vi "ScanDelay_FTIR_PointSpectroscopy.vi"() -> ()   [LabVIEW 2022 SP3] (continued)
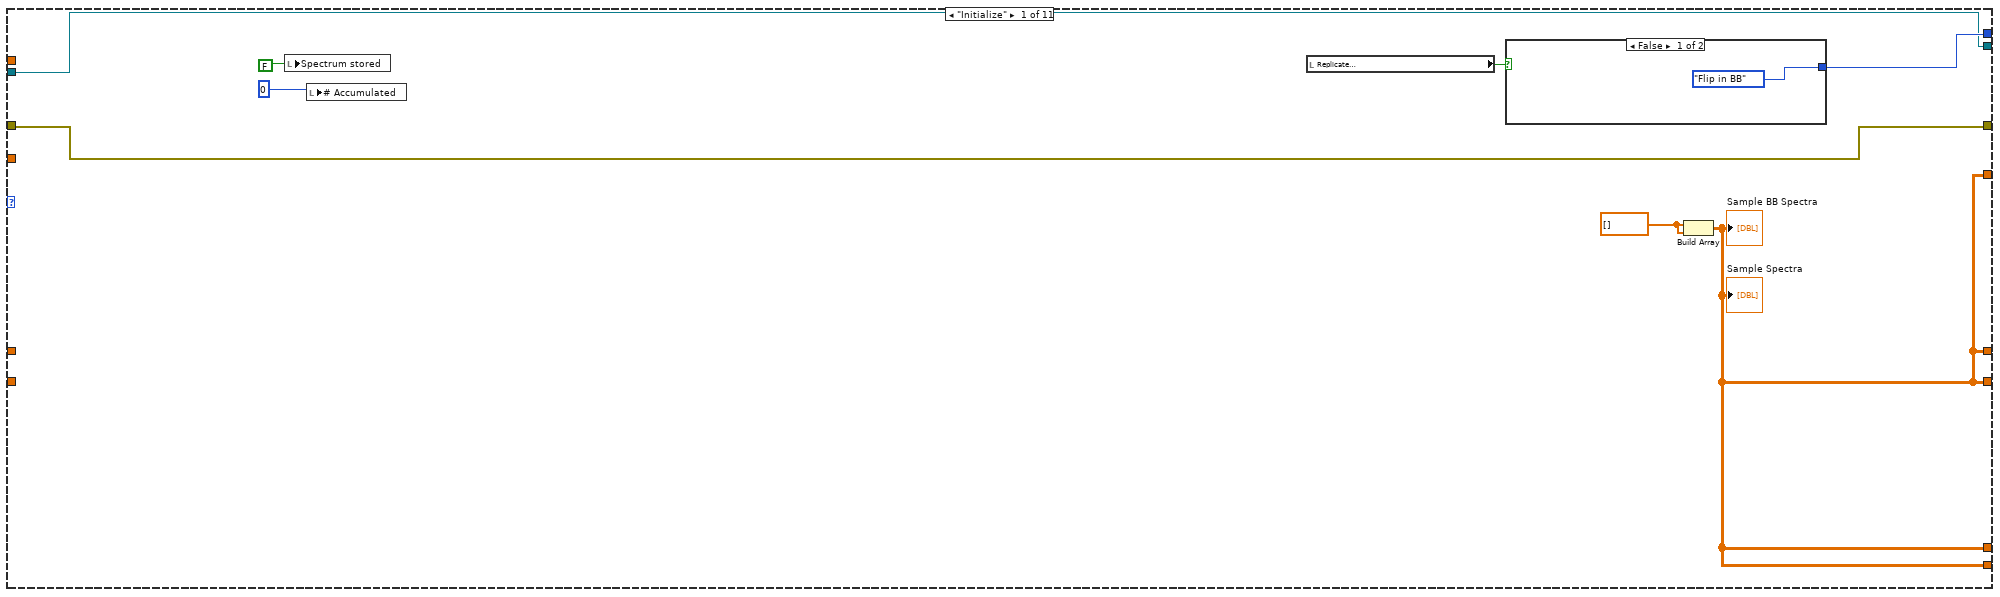
[diagram p3: hidden frame]
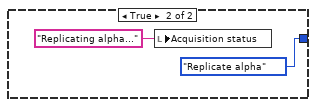
[diagram p4: hidden frame]
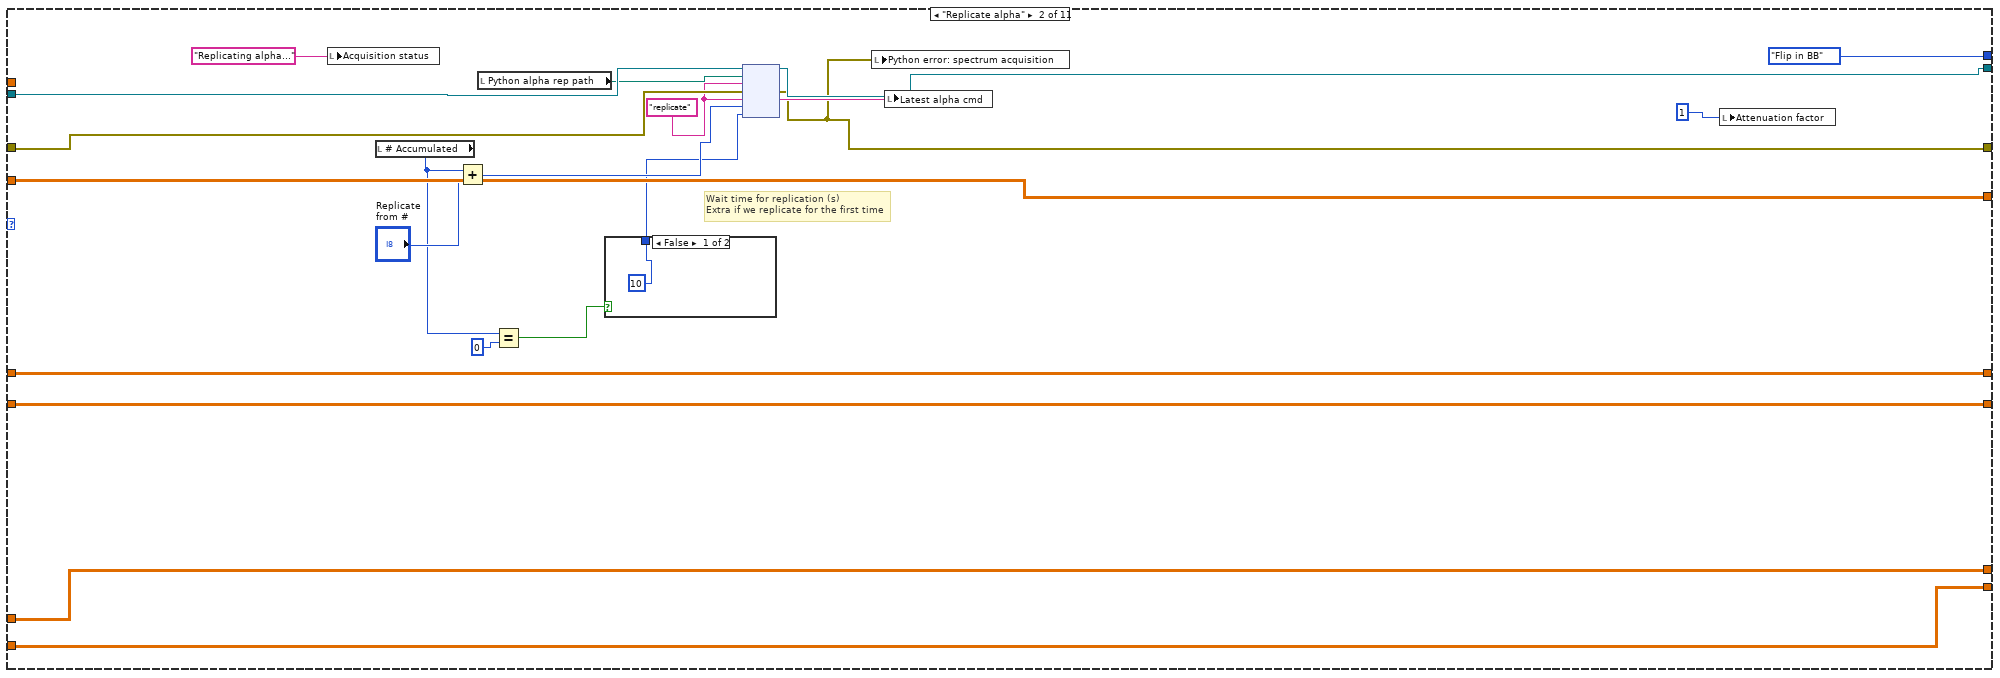
[diagram p5: hidden frame]
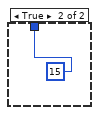
[diagram p6: hidden frame]
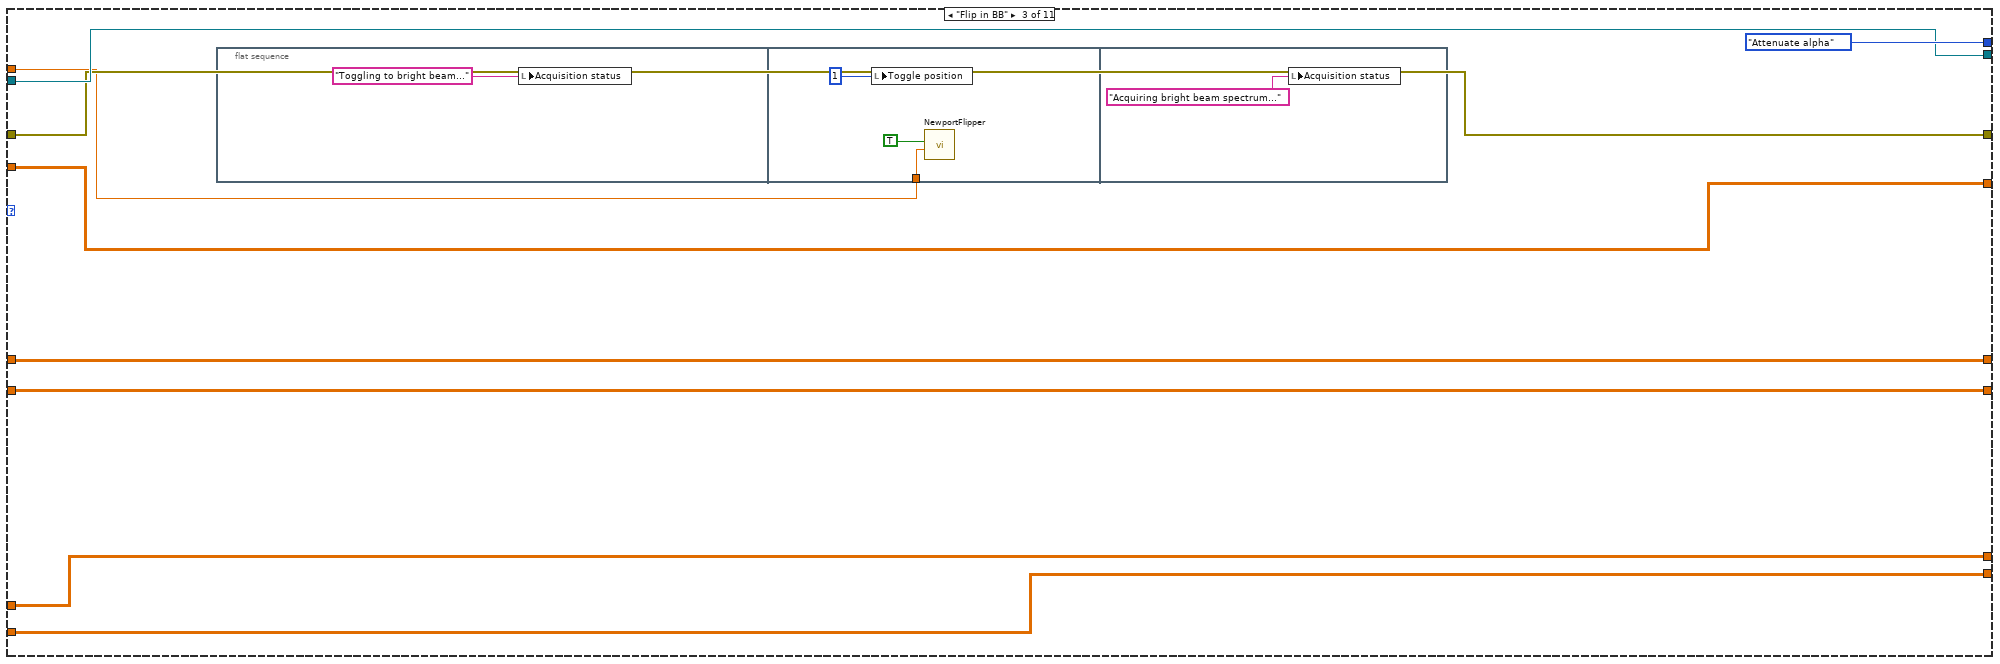
[diagram p7: hidden frame]
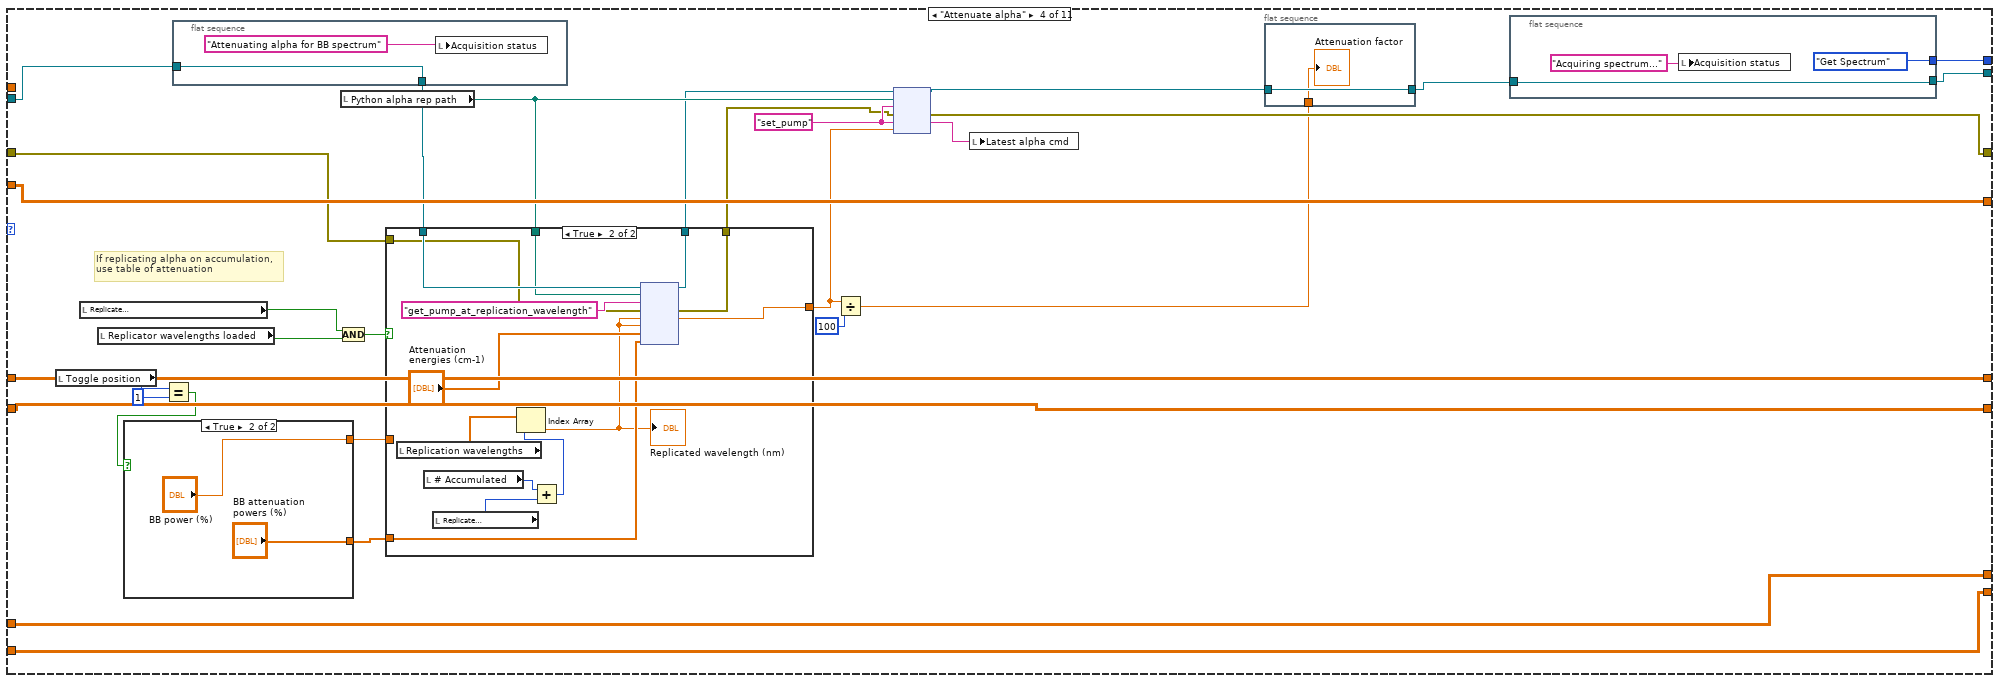
[diagram p8: hidden frame]
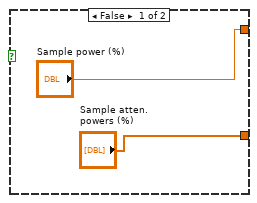
[diagram p9: hidden frame]
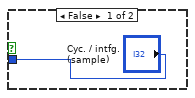
[diagram p11: hidden frame]
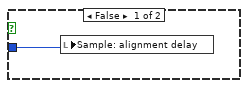
[diagram p13: hidden frame]
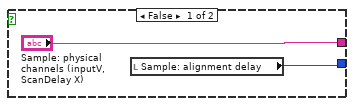
[diagram p14: hidden frame]
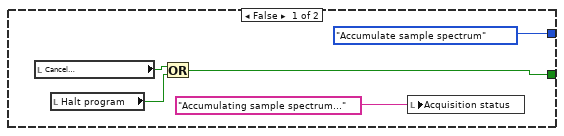
[diagram p16: hidden frame]
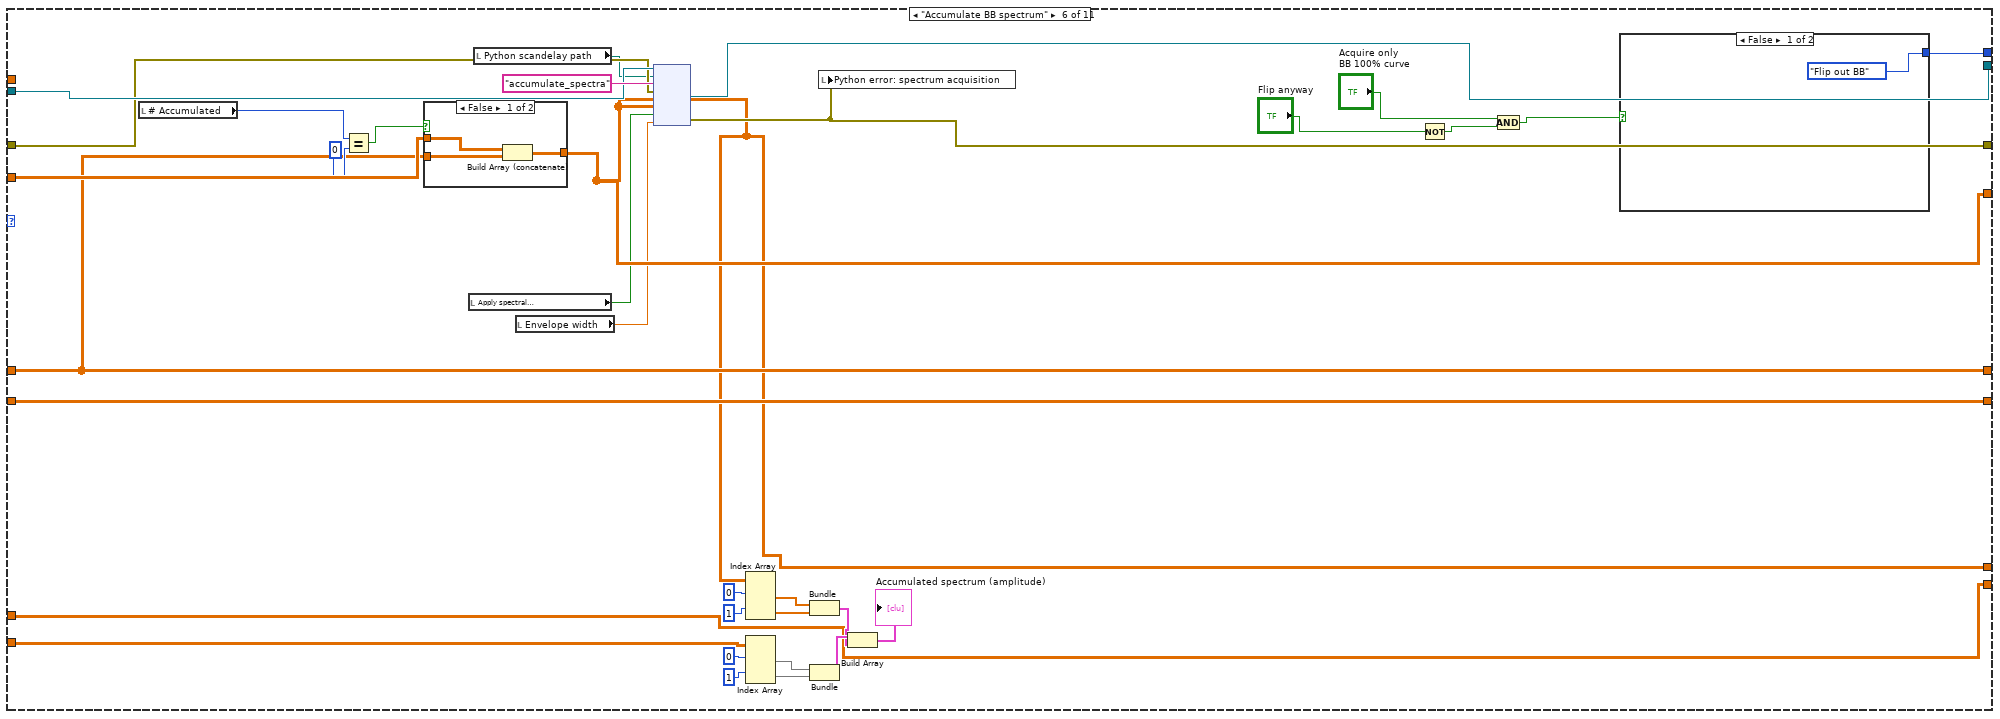
[diagram p17: hidden frame]
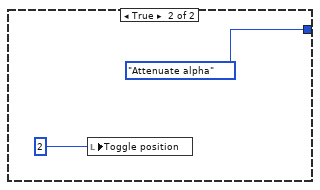
[diagram p18: hidden frame]
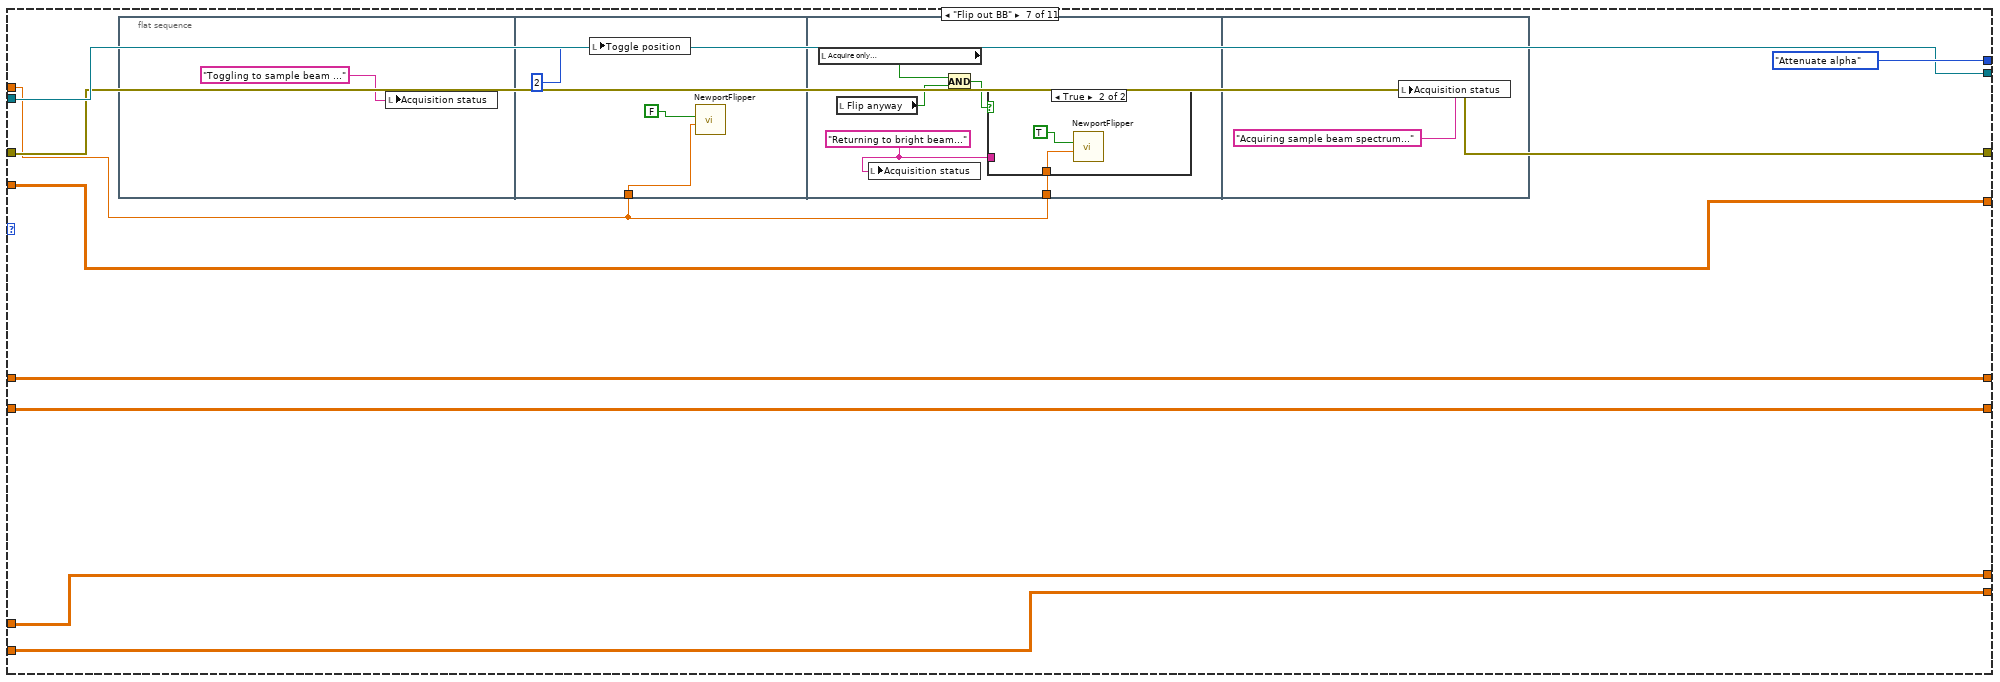
[diagram p20: hidden frame]
            tunnel: w356 -> [w372 w396 w410 w429 w494 w552 w570 w609 w625 w649 w662]
            tunnel: w355 -> [w371 w395 w409 w433 w501 w551 w569 w608 w626 w648 w661]
            tunnel: [w371 w390 w409 w440 w501 w542 w569 w597 w626 w648 w661] -> w354
            tunnel: [w372 w391 w410 w417 w494 w550 w570 w607 w625 w649 w662] -> w353
            tunnel: [w369 w389 w406 w444 w487 w543 w568 w601 w622 w653 w659] -> w352
            tunnel: w350 -> [_ w389 w406 w444 _ w543 w568 w601 w622 w653 w659]
            tunnel: "Toggle pause (ms)" -> [_ _ w403 _ _ _ w565 _ _ _ _]
            tunnel: [w369 w388 w405 w442 w496 w533 w567 w588 w618 w651 w656] -> w348
            tunnel: [w369 w387 w404 w441 w495 w531 w566 w589 w619 w650 w655] -> w347
            tunnel: w346 -> [_ w388 w405 w442 w496 w531 w567 w588 w618 w651 w656]
            tunnel: w345 -> [_ w387 w404 w441 w495 w532 w566 _ w619 w650 w655]
            frame "Initialize" {
              w376 = dbl[] []
              n194 = local write "Spectrum stored"(FALSE) -> ()
              n195 = local write "# Accumulated"(0) -> ()
              n196 = local read "Replicate\nalpha on\naccumulation"() -> (w373:bool)
              n197 = case shown="False" w373 {
                tunnel: [Control_GetSpectrum_BBnorm_AttenuateBB."Flip in BB" Control_GetSpectrum_BBnorm_AttenuateBB."Replicate alpha"] -> w375
                frame False {
                }
                frame True {
                  n198 = local write "Acquisition status"("Replicating alpha...") -> ()
                }
              }
              n199 = Build Array(w376, w376) -> (w369:dbl[][])
              "Sample Spectra" <- w369
              "Sample BB Spectra" <- w369
            }
            frame "Replicate alpha" {
              w393 = "replicate"
              # "Wait time for replication (s)\nExtra if we replicate for the first time"
              n200 = local write "Acquisition status"("Replicating alpha...") -> ()
              n201 = local read "# Accumulated"() -> (w383:i32)
              n202 = Add(x=w383, y="Replicate\nfrom #") -> (x+y=w385:i32)
              n203 = local read "Python alpha rep path"() -> (w394:path)
              n204 = Equal?(x=w383, y=0) -> (x = y?=w382:bool)
              n205 = case shown="False" w382 {
                tunnel: [10 15] -> w381
                frame False {
                }
                frame True {
                }
              }
              n206 = node(w396, w394, w393, w395, w393, w385, w381) -> (w391:refnum<k35>, w390:errorcluster, w392:string)  [unwired: 2 in, 2 out]
              n207 = local write "Python error: spectrum acquisition"(w390) -> ()
              n208 = local write "Latest alpha cmd"(w392) -> ()
              n209 = local write "Attenuation factor"(1) -> ()
            }
            frame "Flip in BB" {
              n210 = flat-sequence {
                tunnel: w403 -> [w413]
                frame #0 {
                  n211 = local write "Acquisition status"("Toggling to bright beam...") -> ()
                }
                frame #1 {
                  n212 = local write "Toggle position"(1) -> ()
                  n213 = call "NewportFlipper.vi"("Settle time (ms)"=w413, "Up/Down"=TRUE) -> ()  [unwired: 10 in]
                }
                frame #2 {
                  n214 = local write "Acquisition status"("Acquiring bright beam spectrum...") -> ()
                }
              }
            }
            frame "Attenuate alpha" {
              w439 = "set_pump"
              # "If replicating alpha on accumulation,\nuse table of attenuation"
              n215 = local read "Toggle position"() -> (w424:i32)
              n216 = local read "Replicate\nalpha on\naccumulation"() -> (w430:bool)
              n217 = local read "Replicator wavelengths loaded"() -> (w435:bool)
              n218 = Equal?(x=w424, y=1) -> (x = y?=w425:bool)
              n219 = case shown="True" w425 {
                tunnel: ["Sample power (%)" "BB power (%)"] -> w422
                tunnel: ["Sample atten.\npowers (%)" "BB attenuation\npowers (%)"] -> w421
                frame False {
                }
                frame True {
                }
              }
              n220 = flat-sequence {
                tunnel: w429 -> [w472]
                tunnel: [w472] -> w428
                frame #0 {
                  n221 = local write "Acquisition status"("Attenuating alpha for BB spectrum") -> ()
                }
              }
              n222 = And(x=w430, y=w435) -> (x .and. y?=w436:bool)
              n223 = local read "Python alpha rep path"() -> (w434:path)
              n224 = case shown="True" w436 {
                tunnel: [w455 w460] -> w420
                tunnel: w428 -> [w457 w467]
                tunnel: w434 -> [_ w466]
                tunnel: w433 -> [w456 w464]
                tunnel: [w457 w463] -> w432
                tunnel: [w456 w462] -> w431
                tunnel: w422 -> [w455 _]
                tunnel: w421 -> [_ w459]
                frame False {
                }
                frame True {
                  n225 = local read "Replication wavelengths"() -> (w469:dbl[])
                  n226 = local read "# Accumulated"() -> (w470:i32)
                  n227 = local read "Replicate\nfrom #"() -> (w471:i8)
                  n228 = Add(x=w470, y=w471) -> (x+y=w468:i32)
                  n229 = Index Array(array=w469, index=w468) -> (element=w458:dbl)
                  "Replicated wavelength (nm)" <- w458
                  n230 = node(w467, w466, "get_pump_at_replication_wavelength", w464, w458, w458, "Attenuation\nenergies (cm-1)", w459) -> (w463:refnum<k35>, w462:errorcluster, w460:dbl)  [unwired: 3 in, 2 out]
                }
              }
              n231 = Divide(x=w420, y=100) -> (x/y=w426:dbl)
              n232 = node(w432, w434, w439, w431, w439, w420) -> (w427:refnum<k35>, w440:errorcluster, w438:string)  [unwired: 1 in, 2 out]
              n233 = local write "Latest alpha cmd"(w438) -> ()
              n234 = flat-sequence {
                tunnel: w427 -> [w454]
                tunnel: [w454] -> w418
                tunnel: w426 -> [w453]
                frame #0 {
                  "Attenuation factor" <- w453
                }
              }
              n235 = flat-sequence {
                tunnel: [Control_GetSpectrum_BBnorm_AttenuateBB."Get Spectrum"] -> w419
                tunnel: w418 -> [w447]
                tunnel: [w447] -> w417
                frame #0 {
                  n236 = local write "Acquisition status"("Acquiring spectrum...") -> ()
                }
              }
            }
            frame "Get Spectrum" {
              n237 = control-ref of="% averaged"() -> (w492:refnum<vi>)
              n238 = control-ref of="Acquisition cycle"() -> (w491:refnum<vi>)
              n239 = control-ref of="Cancel\nacquisition"() -> (w486:refnum<vi>)
              n240 = local read "Toggle position"() -> (w498:i32)
              n241 = control-ref of="Binned interferogram"() -> (w493:refnum<vi>)
              n242 = Equal?(x=w498, y=1) -> (x = y?=w476:bool)
              n243 = case shown="True" w476 {
                tunnel: ["Sample: physical channels (inputV, ScanDelay X)" "Bright beam: physical channels (inputV, ScanDelay X)"] -> w481
                tunnel: [w508 w510] -> w480
                frame False {
                  n244 = local read "Sample: alignment delay"() -> (w508:i32)
                }
                frame True {
                  n245 = local read "Bright beam: alignment delay"() -> (w510:i32)
                }
              }
              n246 = And(x="Optimize\ninterferogram\nalignment", y="Update alignment") -> (x .and. y?=w477:bool)
              n247 = case shown="True" w476 {
                tunnel: ["Cyc. / intfg.\n(sample)" "Cyc. per intfg. (BB)"] -> w475
                frame False {
                }
                frame True {
                }
              }
              n248 = call "ScanDelay_FTIR_GetSpectrum_Aligning.vi"("Cancel? External"=w486, "% averaged (external)"=w492, "Binned interferogram (external)"=w493, "Python refnum in"=w494, "Optimize\ninterferogram\ndelay"="Optimize\ninterferogram\nalignment", "Acquisition cycle (external)"=w491, "Gain"=1.0, "Displacement\n calibration  factor"="Delay calibratior\nfactor (ps/V)", "Channels to read (input V, ScanDelay)"=w481, "Acquisitions per interferogram"=w475, "Time per\nacquisition (s)"="Time per\nacquisition (s)", "Sampling rate"="Sampling rate", "Delay estimation (pts)"=w480) -> ("Output spectrum"=w487:dbl[][], "Best delay"=w482:i32)  [unwired: 1 in]
              n249 = case shown="True" w477 {
                tunnel: w482 -> [_ w505]
                tunnel: w476 -> [_ w504]
                frame False {
                }
                frame True {
                  # "Update our optimal delay only if we are actively optimizing"
                  n250 = case shown="True" w504 {
                    tunnel: w505 -> [w506 w507]
                    frame False {
                      n251 = local write "Sample: alignment delay"(w506) -> ()
                    }
                    frame True {
                      n252 = local write "Bright beam: alignment delay"(w507) -> ()
                    }
                  }
                }
              }
              n253 = case shown="True" w476 {
                tunnel: [Control_GetSpectrum_BBnorm_AttenuateBB."Accumulate sample spectrum" Control_GetSpectrum_BBnorm_AttenuateBB."Accumulate BB spectrum"] -> w485
                tunnel: w487 -> [_ _]
                tunnel: [w514 w519] -> w483
                frame False {
                  n254 = local read "Cancel\nacquisition"() -> (w515:bool)
                  n255 = local read "Halt program"() -> (w516:bool)
                  n256 = Or(x=w515, y=w516) -> (x .or. y?=w514:bool)
                  n257 = local write "Acquisition status"("Accumulating sample spectrum...") -> ()
                }
                frame True {
                  n258 = local read "Cancel\nacquisition"() -> (w521:bool)
                  n259 = local read "Halt program"() -> (w520:bool)
                  n260 = Or(x=w521, y=w520) -> (x .or. y?=w519:bool)
                  n261 = local write "Acquisition status"("Accumulating bright beam spectrum...") -> ()
                }
              }
              n262 = case shown="True" w483 {
                tunnel: w485 -> [w512 _]
                tunnel: [w512 Control_GetSpectrum_BBnorm_AttenuateBB."Done"] -> w484
                frame False {
                }
                frame True {
                }
              }
            }
            frame "Accumulate BB spectrum" {
              n263 = local read "# Accumulated"() -> (w556:i32)
              n264 = Equal?(x=w556, y=0) -> (x = y?=w554:bool)
              n265 = case shown="False" w554 {
                tunnel: w543 -> [w562 w564]
                tunnel: w557 -> [w563 _]
                tunnel: [w561 w564] -> w548
                frame False {
                  n266 = Build Array (concatenate)(w563, w562) -> (w561:dbl[][])
                }
                frame True {
                }
              }
              n267 = local read "Apply spectral\nenvelope"() -> (w530:bool)
              n268 = local read "Python scandelay path"() -> (w549:path)
              n269 = local read "Envelope width"() -> (w529:dbl)
              n270 = node(w552, w549, "accumulate_spectra", w551, w548, w548, w530, w529) -> (w550:refnum<k35>, w542:errorcluster, w533:dbl[][])  [unwired: 3 in, 2 out]
              n271 = Index Array(array=w533, index (row) #1=0, index (row) #2=1) -> (element #1=w545:dbl[], element #2=w544:dbl[])  [unwired: 2 in]
              n272 = Index Array(array=w532, index (row) #1=0, index (row) #2=1) -> (element #1=w539:dbl[], element #2=w538:dbl[])  [unwired: 2 in]
              n273 = Bundle("Output spectrum"=w545, "Output spectrum"=w544) -> (w535:T1)  [unwired: 1 in]
              n274 = Bundle("Output spectrum"=w539, "Output spectrum"=w538) -> (w536:T1)  [unwired: 1 in]
              n275 = local write "Python error: spectrum acquisition"(w542) -> ()
              n276 = Build Array(w536, w535) -> (→"Accumulated spectrum (amplitude)":T3)
              n277 = Not(x="Flip anyway") -> (.not. x?=w526:bool)
              n278 = And(x="Acquire only\nBB 100% curve", y=w526) -> (x .and. y?=w525:bool)
              n279 = case shown="False" w525 {
                tunnel: [Control_GetSpectrum_BBnorm_AttenuateBB."Flip out BB" Control_GetSpectrum_BBnorm_AttenuateBB."Attenuate alpha"] -> w528
                frame False {
                }
                frame True {
                  n280 = local write "Toggle position"(2) -> ()
                }
              }
            }
            frame "Flip out BB" {
              n281 = flat-sequence {
                tunnel: w565 -> [w576]
                tunnel: w565 -> [w582]
                frame #0 {
                  n282 = local write "Acquisition status"("Toggling to sample beam ...") -> ()
                }
                frame #1 {
                  n283 = local write "Toggle position"(2) -> ()
                  n284 = call "NewportFlipper.vi"("Settle time (ms)"=w576, "Up/Down"=FALSE) -> ()  [unwired: 10 in]
                }
                frame #2 {
                  w578 = "Returning to bright beam..."
                  n285 = local read "Acquire only\nBB 100% curve"() -> (w581:bool)
                  n286 = local read "Flip anyway"() -> (w580:bool)
                  n287 = local write "Acquisition status"(w578) -> ()
                  n288 = And(x=w581, y=w580) -> (x .and. y?=w579:bool)
                  n289 = case shown="True" w579 {
                    tunnel: w582 -> [_ w583]
                    tunnel: w578 -> [_ _]
                    frame False {
                    }
                    frame True {
                      n290 = call "NewportFlipper.vi"("Settle time (ms)"=w583, "Up/Down"=TRUE) -> ()  [unwired: 10 in]
                    }
                  }
                }
                frame #3 {
                  n291 = local write "Acquisition status"("Acquiring sample beam spectrum...") -> ()
                }
              }
            }
            frame "Accumulate sample spectrum" {
              (unwired) 0
              n292 = local read "# Accumulated"() -> (w613:i32)
              n293 = Equal?(x=w613, y=0) -> (x = y?=w611:bool)
              n294 = case shown="True" w611 {
                tunnel: w601 -> [w615 w617]
                tunnel: w599 -> [w616 _]
                tunnel: [w614 w617] -> w598
                frame False {
                  n295 = Build Array (concatenate)(w616, w615) -> (w614:dbl[][])
                }
                frame True {
                }
              }
              n296 = local read "Apply spectral\nenvelope"() -> (w587:bool)
              n297 = local read "Python scandelay path"() -> (w606:path)
              n298 = local read "Envelope width"() -> (w586:dbl)
              n299 = node(w609, w606, "accumulate_spectra", w608, w598, w598, w587, w586) -> (w607:refnum<k35>, w597:errorcluster, w589:dbl[][])  [unwired: 3 in, 2 out]
              n300 = local write "Python error: spectrum acquisition"(w597) -> ()
              n301 = Index Array(array=w589, index (row) #1=0, index (row) #2=1) -> (element #1=w603:dbl[], element #2=w602:dbl[])  [unwired: 2 in]
              n302 = Index Array(array=w588, index (row) #2=1) -> (element #1=w594:dbl[], element #2=w593:dbl[])  [unwired: 3 in]
              n303 = Bundle("Output spectrum"=w603, "Output spectrum"=w602) -> (w596:T1)  [unwired: 1 in]
              n304 = Bundle("Output spectrum"=w594, "Output spectrum"=w593) -> (w592:T1)  [unwired: 1 in]
              n305 = Build Array(w596, w592) -> (w590:T3)
              n306 = property on="Accumulated spectrum (amplitude)" class="XYGraph (strict)"("Value"=w590) -> ()  [unwired: 2 in, 2 out]
            }
            frame "Assess accumulation" {
              n307 = flat-sequence {
                tunnel: [w631] -> w624
                tunnel: w621 -> [w630]
                tunnel: w620 -> [w629]
                tunnel: w619 -> [w627]
                tunnel: w618 -> [w628]
                tunnel: w624 -> [w633]
                tunnel: [w637] -> w623
                frame #0 {
                  n308 = local read "# Accumulated"() -> (w632:i32)
                  n309 = local write "Accumulated sample spectrum"(w627) -> ()
                  n310 = Increment(x=w632) -> (x+1=w631:i32)
                  n311 = local write "Accumulated sample BB spectrum"(w628) -> ()
                  n312 = local write "Sample Spectra"(w629) -> ()
                  n313 = local write "Sample BB Spectra"(w630) -> ()
                  n314 = local write "# Accumulated"(w631) -> ()
                }
                frame #1 {
                  n315 = local read "Accumulate to #"() -> (w634:i32)
                  n316 = property on="BB-reference spectrum" class="Bool (strict)"("Val(Sgnl)"=TRUE) -> ()  [unwired: 2 in, 2 out]
                  n317 = Less Or Equal?(x=w634, y=w633) -> (x <= y?=w635:bool)
                  n318 = case shown="False" w635 {
                    tunnel: [w638 Control_GetSpectrum_BBnorm_AttenuateBB."Finalize"] -> w637
                    frame False {
                      n319 = local read "Replicate\nalpha on\naccumulation"() -> (w639:bool)
                      n320 = case shown="True" w639 {
                        tunnel: [Control_GetSpectrum_BBnorm_AttenuateBB."Flip in BB" Control_GetSpectrum_BBnorm_AttenuateBB."Replicate alpha"] -> w638
                        frame False {
                          n321 = local write "Acquisition status"("Toggling to bright beam") -> ()
                        }
                        frame True {
                          n322 = local write "Acquisition status"("Replicating alpha...") -> ()
                        }
                      }
                    }
                    frame True {
                    }
                  }
                }
              }
            }
            frame "Finalize" {
              n323 = local write "Spectrum stored"(TRUE) -> ()
            }
            frame "Done" {
              w654 = FALSE
              n324 = local write "Acquire spectrum"(w654) -> ()
              n325 = local write "Cancel\nacquisition"(w654) -> ()
            }
          }
          n326 = Wait (ms)(milliseconds to wait=5) -> ()  [unwired: 1 out]
        }
      }
      event Timeout {
        n327 = event-data() -> ()  [unwired: 1 in, 3 out]
        n328 = Wait (ms)(milliseconds to wait=w665) -> ()  [unwired: 1 out]
      }
    }
    n329 = Wait (ms)(milliseconds to wait=5) -> ()  [unwired: 1 out]
    n330 = local read "Halt program"() -> (w333:bool)
    "Acquisition status" <- "Ready to acquire spectrum"
  }
  n331 = Close Python Session(session in=w13, error in=w12) -> (11:w9:errorcluster)
  n332 = local write "Python error: activity loop"(w9) -> ()
  n333 = Close Python Session(session in=w3, error in=w2) -> ()  [unwired: 1 out]
